vi "Main.vi"() -> ()   [LabVIEW 2020]
uses:
  System.Windows.Forms
  Global_Variable/Global.vi
  Database/Global1.vi
  <userlib>/_MGI/Menu Building/MenuTypes/MenuStrip/MGI_MenuStrip.lvclass
  <userlib>/_MGI/Menu Building/MenuItemStatusChange/MGI_MenuItemStatusChange.lvclass
  S7/S7.lvlib
panel:
  in  "Result":string[][](table)
  out "传感器码":string
  out "上序状态":string
  in  "Andon":enum32{"未选择", "缺料报警", "质量报警", "故障报警"}(radio)
  out "PLC":bool
  in  "菜单":refnum<k24>(container)
  out "逆向空载":bool
  out "试验计时":u16
  out "生产数量":i32
  out "合格数量":i32
  out "userStatus":string caption="用户状态"
  out "userName":string caption="用户名"
  out "connectionMode":string caption="联机类型"
  out "产品型号":string
  out "手柄开启力":bool
  out "手柄锁紧力":bool
  out "振动NVH":bool
  out "备用试验1":bool
  out "备用试验2":bool
  out "手柄保持力":bool caption="管柱保持力"
  out "锁紧/开启":bool
  out "手柄推拉力":bool caption="管柱推拉力"
  in  "更换产品":refnum<vi>
  out "提示信息":string
  out "错误":bool
  out "时间字符串":string
  out "日期字符串":string
  out "自动":bool
  # "滑移力检测"
  # "上序状态"
  # "试验项目"
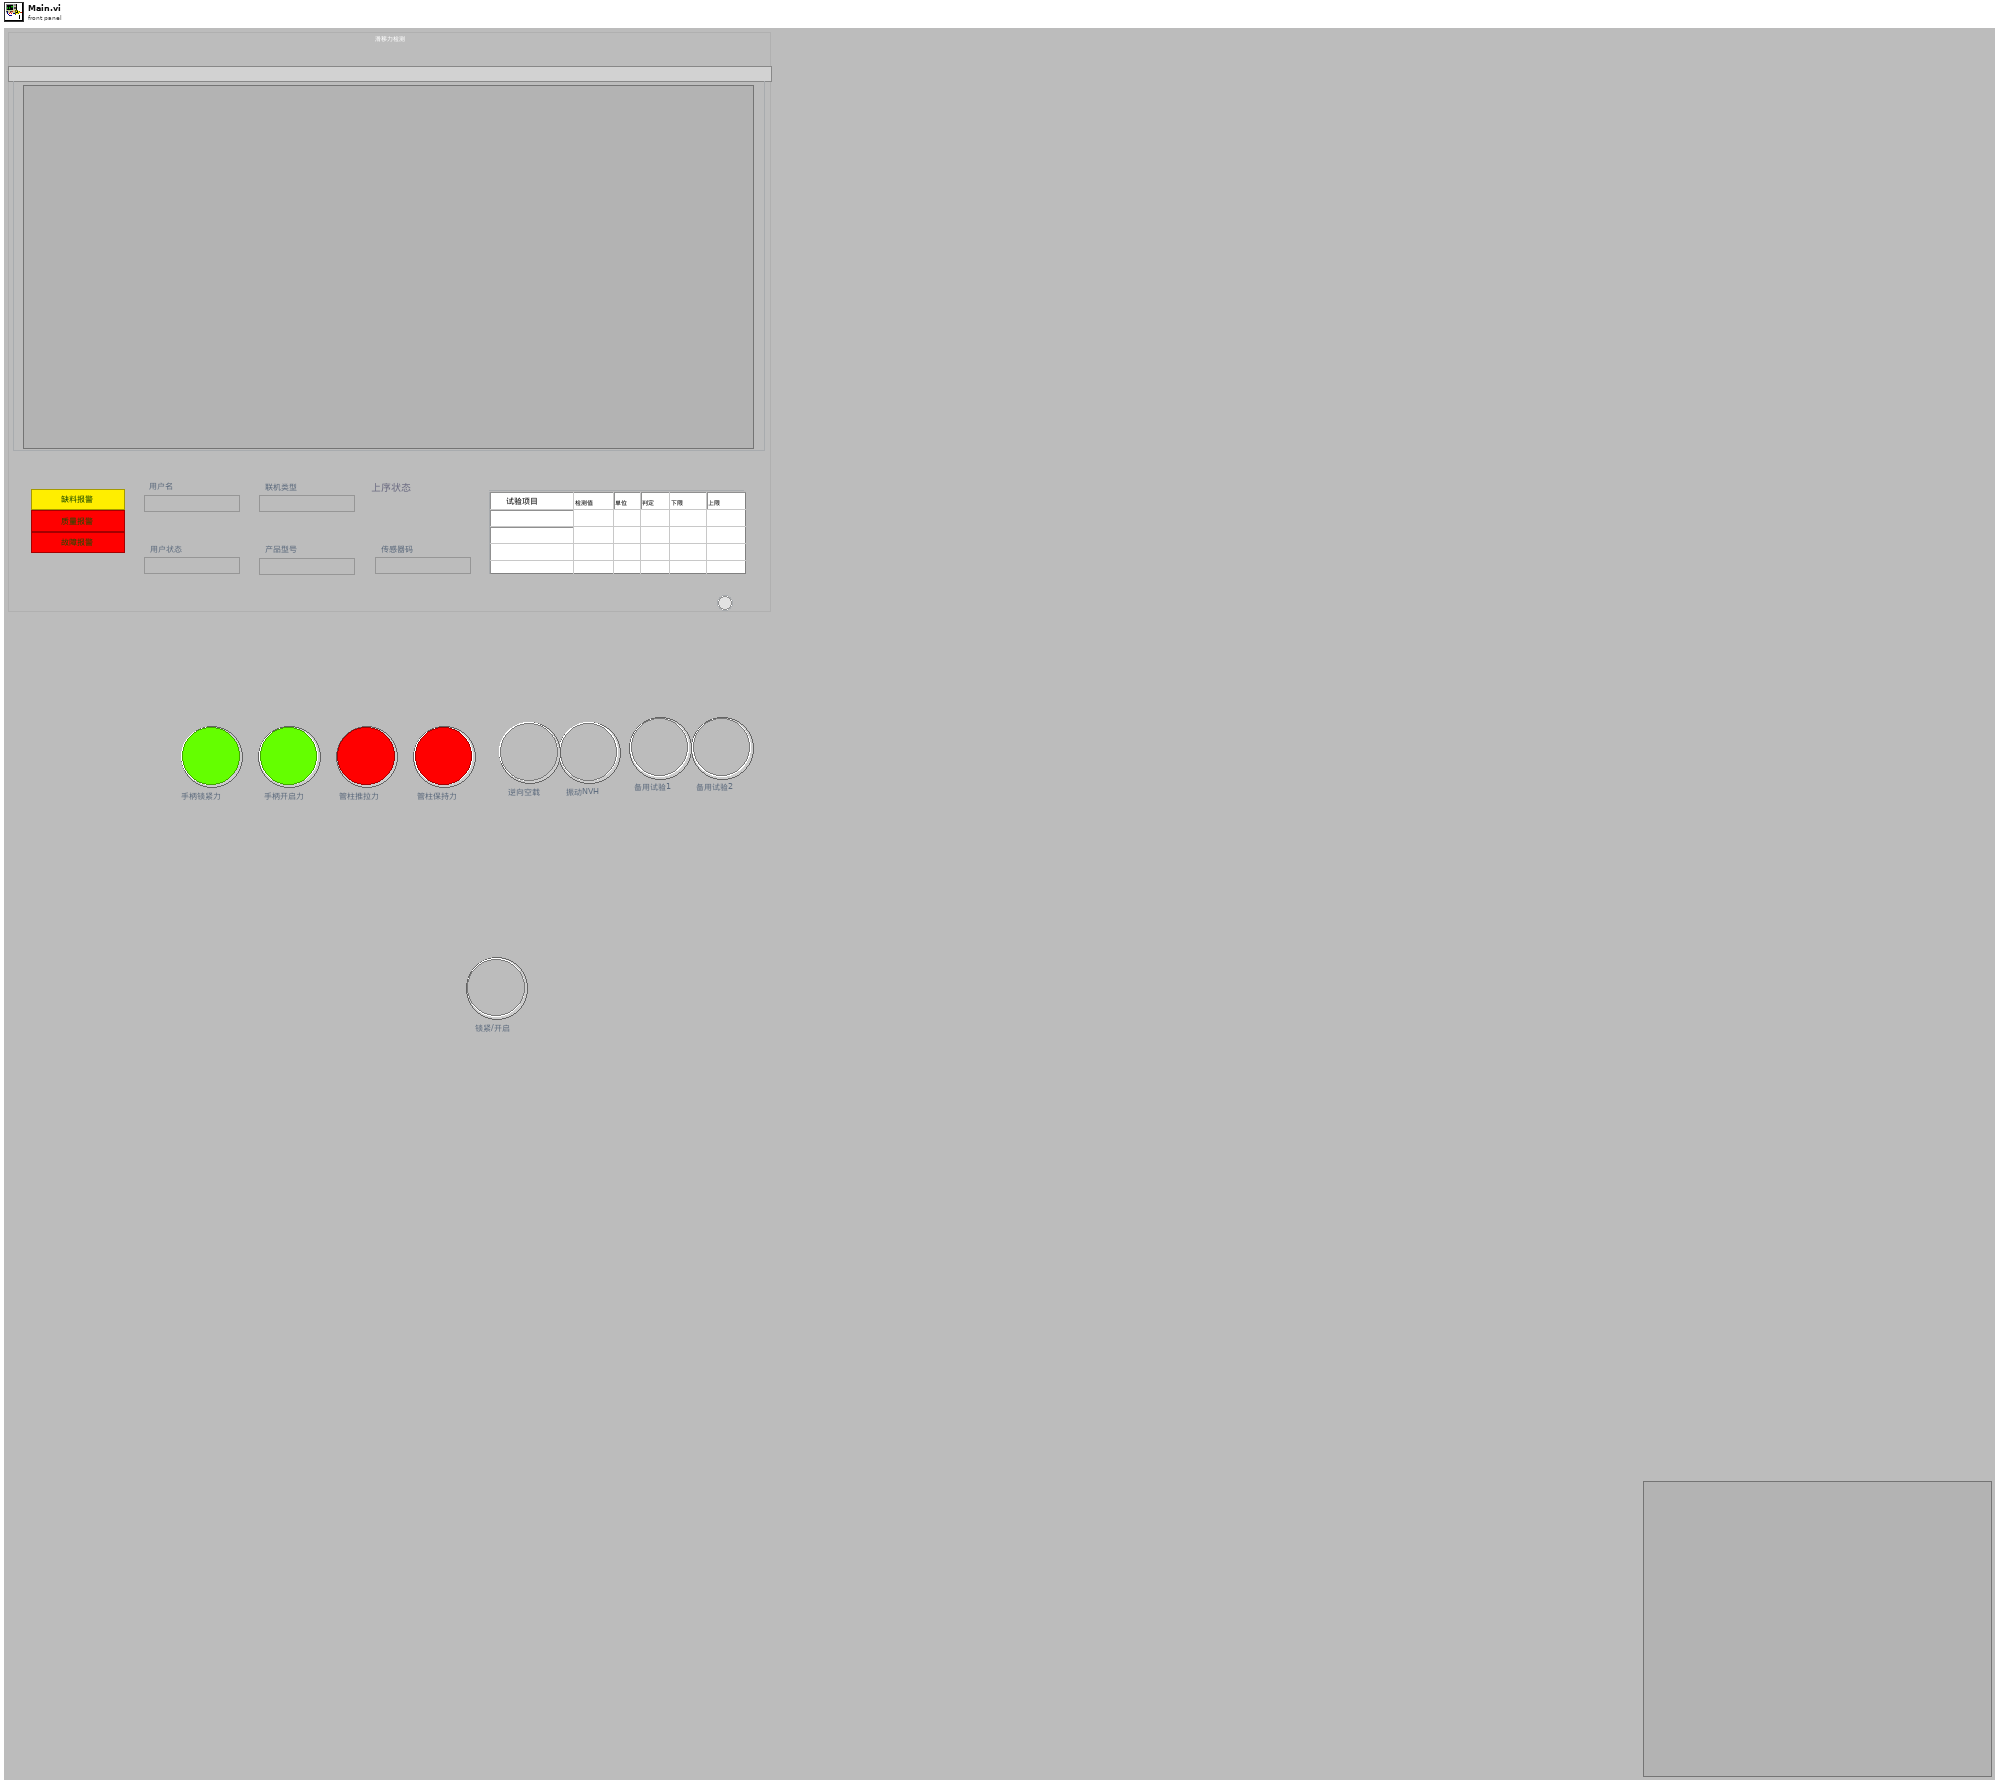
[diagram p1: front panel]
types:
  T1 = typedef "S7.lvlib/Broadcast Events--cluster.ctl" = cluster{"Module Did Init":refnum<user-event>, "Status Updated":refnum<user-event>, "Error Reported":refnum<user-event>, "Module Did Stop":refnum<user-event>, "Update Module Execution Status":refnum<user-event>}
  T2 = enum32{"Invalid", "Standard", "Closed", "Hidden", "Minimized", "Maximized"}
  T3 = cluster{"设备名称":string, "操作人员":string, "设备状态":enum16{"设备离线", "设备正常", "设备缺料", "设备故障", "质量报警"}, "附加信息":string}
  T4 = enum32{"invalid app kind", "Development System", "Run Time System", "Student Edition", "Embedded LabVIEW", "Evaluation", "Custom"}
  T5 = cluster{"用户编号":string, "用户名":string, "用户密码(密文)":string, "用户权限":string}
  T6 = cluster{"Core":cluster{"Current VI Reference":refnum<vi>, "Close Panel on Exit?":bool}, "Your Boolean data":bool, "Your string data":string}
  T7 = cluster{"Current VI Reference":refnum<vi>, "Close Panel on Exit?":bool}
  T8 = cluster{"设备名称":string, "用户名":string, "设备状态":enum16{"设备离线", "设备正常", "设备缺料", "设备故障", "质量报警"}, "附加信息":string}
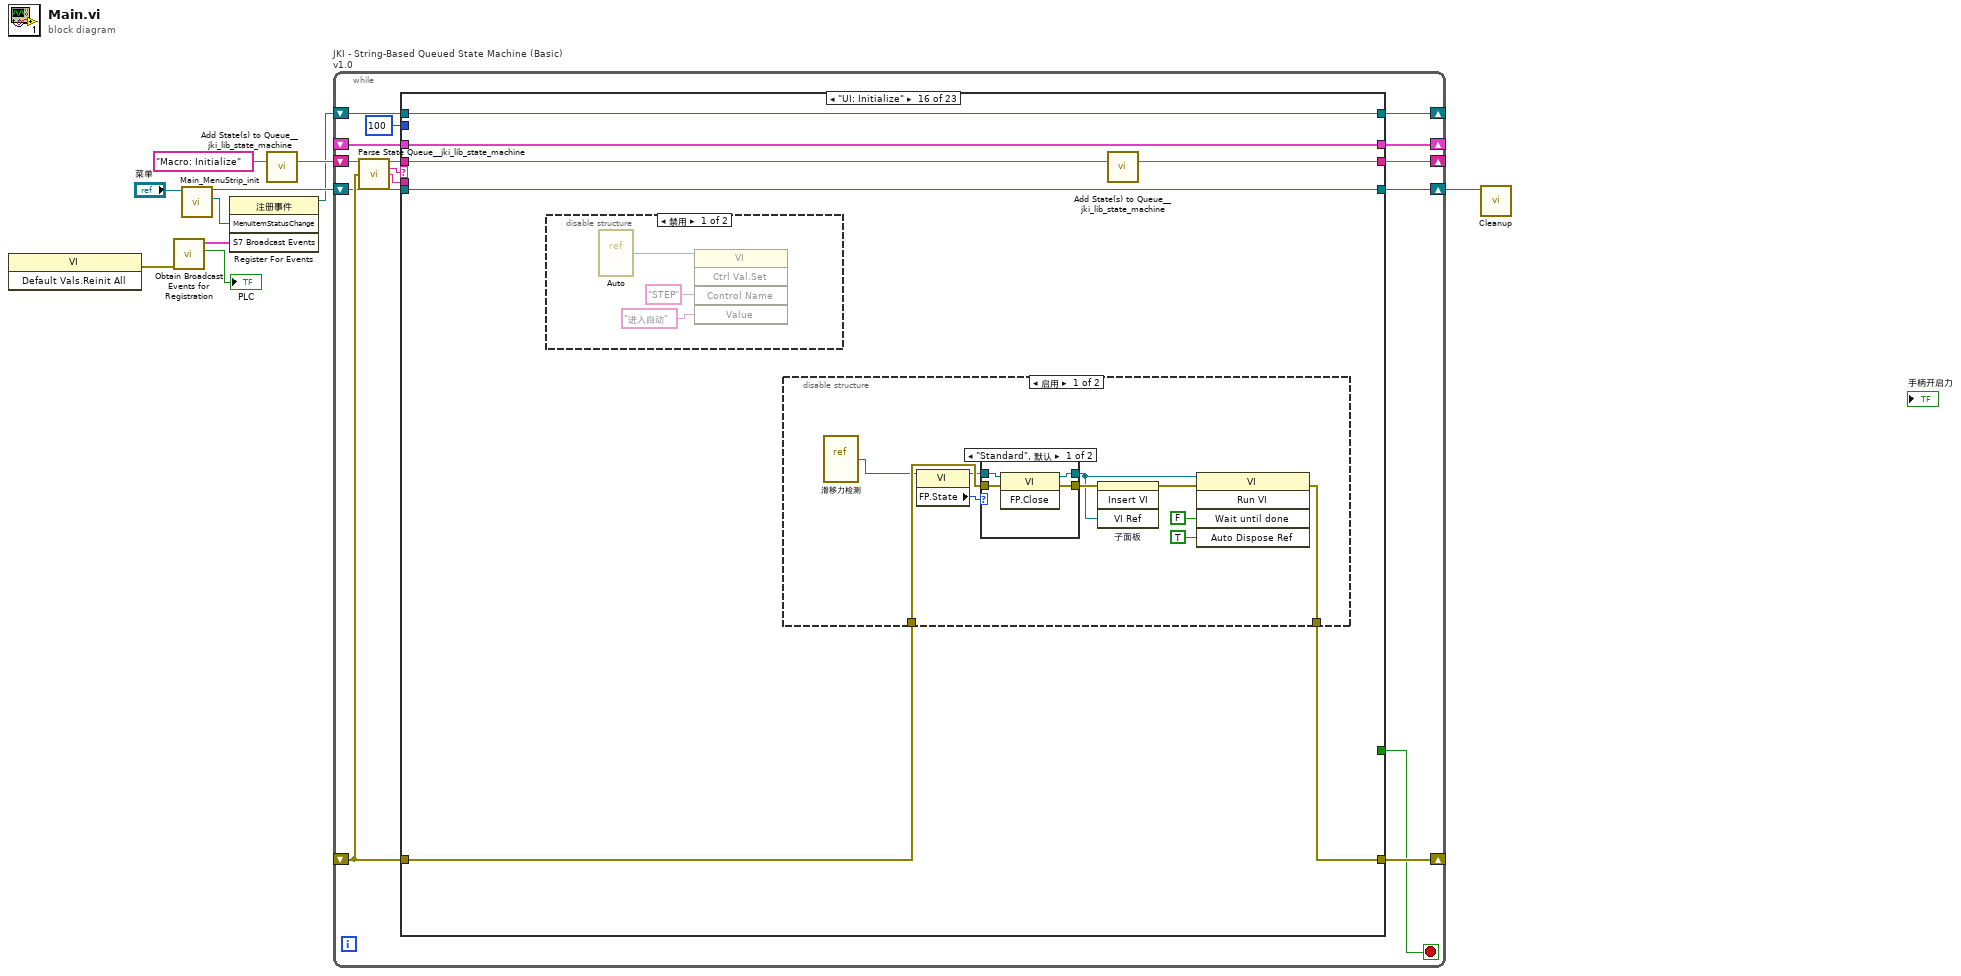
[diagram p0: block diagram]
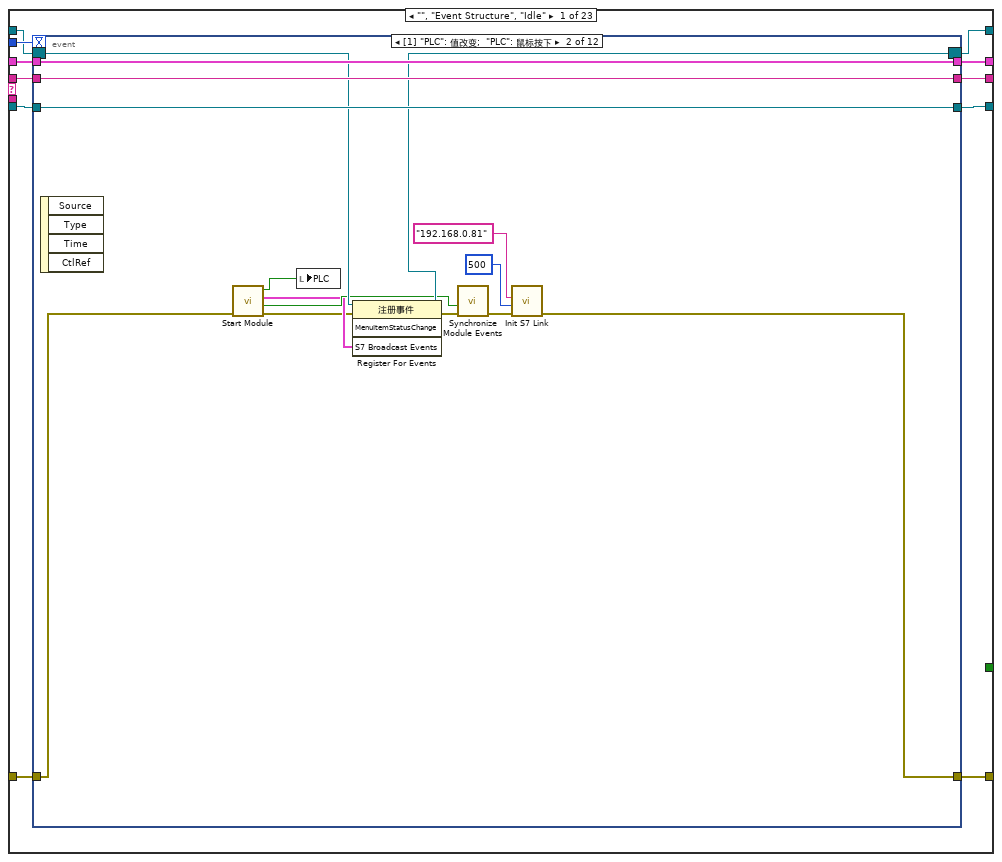
[diagram p2: hidden frame]
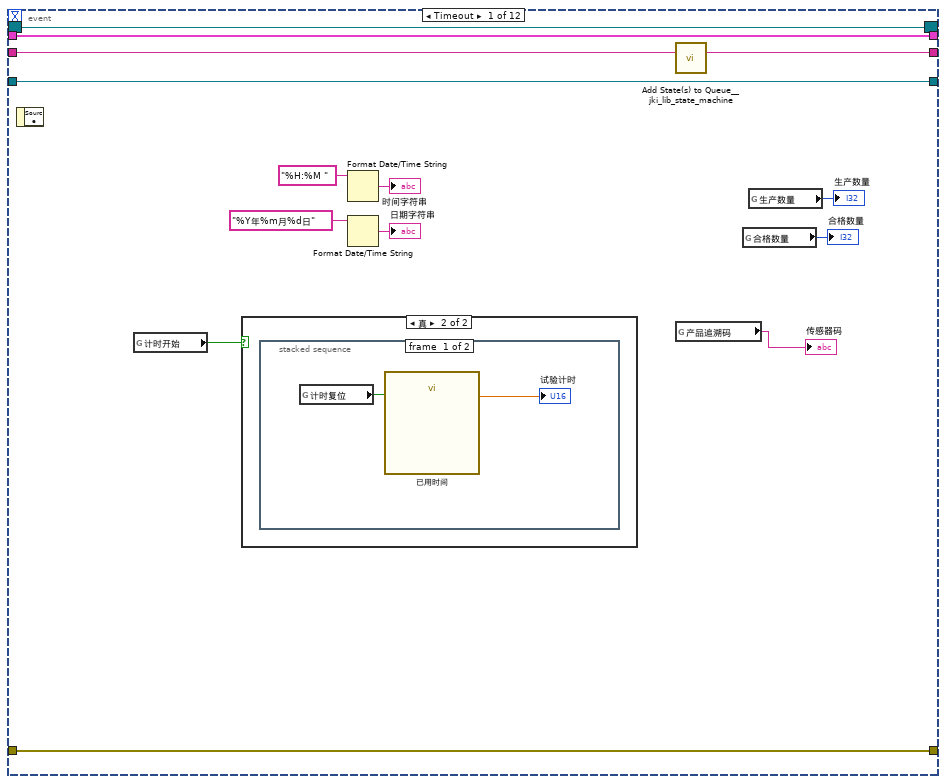
[diagram p3: hidden frame]
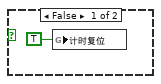
[diagram p4: hidden frame]
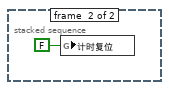
[diagram p5: hidden frame]
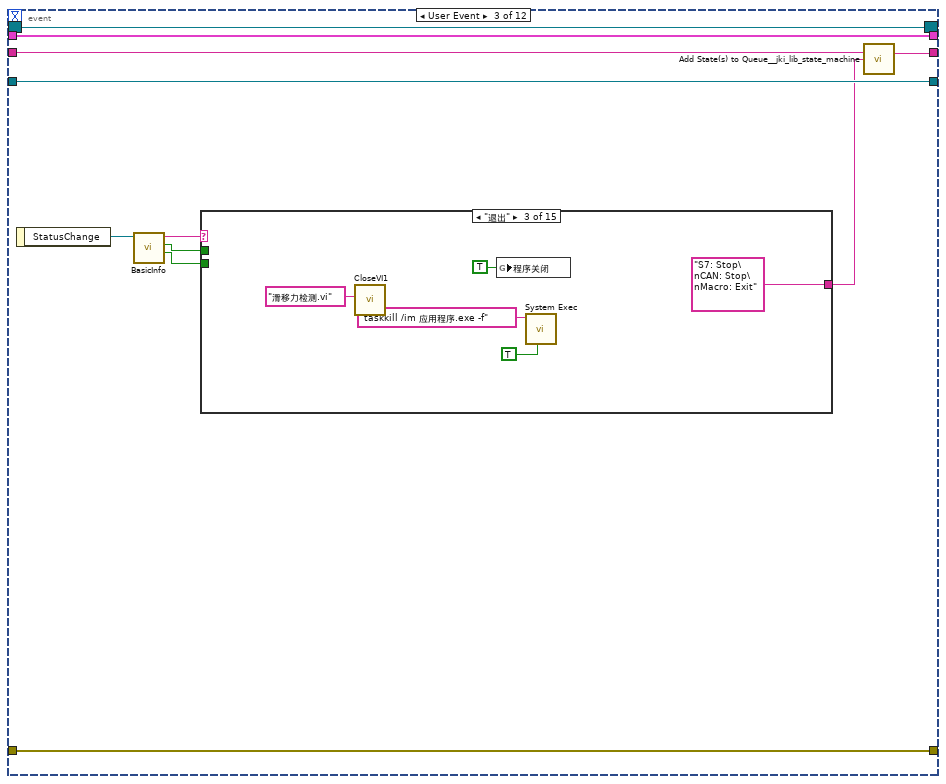
[diagram p6: hidden frame]
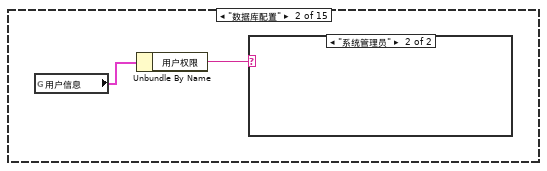
[diagram p8: hidden frame]
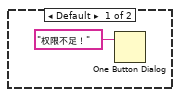
[diagram p9: hidden frame]
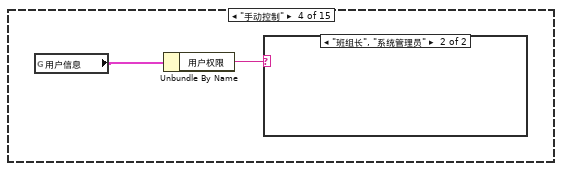
[diagram p10: hidden frame]
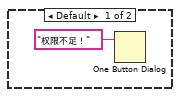
[diagram p11: hidden frame]
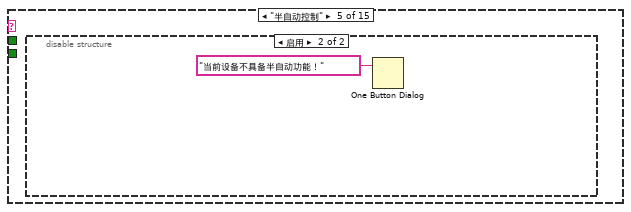
[diagram p12: hidden frame]
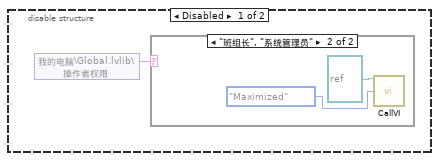
[diagram p13: hidden frame]
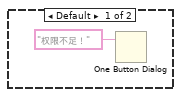
[diagram p14: hidden frame]
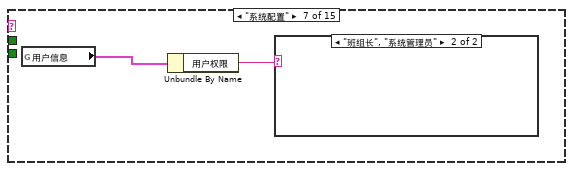
[diagram p16: hidden frame]
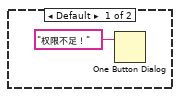
[diagram p17: hidden frame]
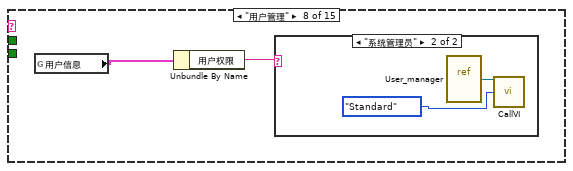
[diagram p18: hidden frame]
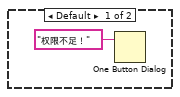
[diagram p19: hidden frame]
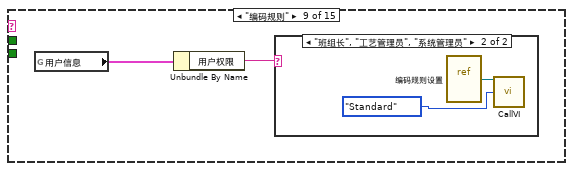
[diagram p20: hidden frame]
diagram:
  n1 = invoke class="VI" method="Default Vals.Reinit All"() -> (error out=w3:errorcluster)  [unwired: 3 in, 2 out]
  n2 = call "Obtain Broadcast Events for Registration.vi"("error in (no error)"=w3) -> ("Already running?"=→"PLC":bool, "S7 Broadcast Events"=w5:T1)  [unwired: 8 in, 1 out]
  n3 = call "Main_MenuStrip_init.vi"("MenuStrip"="菜单") -> ("MenuItemStatusChange"=w2:refnum<user-event>, "Menu out"=w7:refnum<class "MGI_MenuStrip.lvclass">)  [unwired: 9 in]
  n4 = register-events(w2, w5) -> (reference out=w1:refnum<event-registration>)  [unwired: 2 in, 1 out]
  n5 = call <vilib>:"Add State(s) to Queue__jki_lib_state_machine.vi"("State(s) in (\"\")"="Macro: Initialize") -> ("States Out"=w10:string)  [unwired: 14 in]
  n6 = while "JKI - String-Based Queued State Machine (Basic) v1.0" {
    shift-right: [w19] -> _
    shift-left: _ -> [w18]
    shift-right: [w21] -> _
    shift-left: _ -> [w16]
    shift-right: [w20] -> _
    shift-left: w10 -> [w22]
    shift-right: [w14] -> w6
    shift-left: w7 -> [w15]
    shift-right: [w12] -> _
    shift-left: w1 -> [w11]
    stop <- w13 stop-if-true
    n7 = call <vilib>:"Parse State Queue__jki_lib_state_machine.vi"("State Queue"=w22, "Error In (no error)"=w16) -> ("Remaining States"=w24:string, "Current State"=w25:string, "Arguments"=w23:string)  [unwired: 11 in]
    n8 = case shown="\"UI: Initialize\"" w25 {
      selector: w25 -> [_ _ w243 _ _ _ _ _ _ _ _ _ _ _ _ _ _ _ _ _ _ _ _]
      tunnel: w24 -> [w36 w240 w247 w267 w275 w282 w288 w292 w298 w304 w310 w319 w330 w338 w344 w351 w378 w417 w425 w438 w466 w473 w485]
      tunnel: w23 -> [_ _ _ _ _ _ _ _ _ _ _ _ _ _ _ _ _ _ w420 w432 _ _ _]
      tunnel: w18 -> [w34 w237 w245 w258 w272 w280 w285 w293 w301 w307 w313 w316 _ w333 w341 w349 w376 w414 w423 w434 w463 w470 w482]
      tunnel: [w33 w238 w249 w264 errorcluster {"status"=FALSE, "code"=0, "source"=""} ("error out") w279 w286 w290 w296 w303 w309 w317 w327 w334 w342 w348 w374 w415 w421 w435 w464 w471 w483] -> w21
      tunnel: w16 -> [w32 w238 w248 w264 w271 w279 w286 w290 w297 w303 w309 w317 w327 w335 w342 w345 w374 w415 w422 w436 w464 w471 w483]
      tunnel: [w35 w239 w246 w266 w274 w281 w287 w292 w299 w305 w311 w318 w329 w337 w343 w350 w377 w416 w424 w437 w465 w472 w484] -> w20
      tunnel: [w31 w237 w245 w265 w272 w280 w285 w293 w301 w307 w313 w316 w328 w333 w341 w349 w376 w414 w423 w434 w463 w470 w482] -> w19
      tunnel: 100 ("Timeout") -> [w30 _ _ _ _ _ _ _ _ _ _ _ _ _ _ _ _ _ _ _ _ _ _]
      tunnel: w15 -> [w29 w236 w242 w255 w269 w278 w284 w291 w300 w306 w312 w315 w321 w332 w340 w347 w375 w413 w419 w431 w462 w468 w475]
      tunnel: [w28 w236 w242 w255 w269 w278 w284 w291 w300 w306 w312 w315 w321 w332 w340 w347 w375 w413 w419 w431 w462 w468 w475] -> w14
      tunnel: [_ _ _ _ _ TRUE _ _ _ _ _ _ _ _ _ _ _ _ _ _ _ _ _] -> w13
      tunnel: [w26 w235 w241 w254 w268 w276 w283 w294 w295 w302 w308 w314 w322 w331 w339 w346 w373 w412 w418 w430 w461 w467 w474] -> w12
      tunnel: w11 -> [w27 w235 w241 w254 w268 w276 w283 w294 w295 w302 w308 w314 w322 w331 w339 w346 w373 w412 w418 w430 w461 w467 w474]
      frame "", "Event Structure", "Idle" {
        n9 = event shown="[1] \"PLC\": 值改变;  \"PLC\": 鼠标按下" {
          selector: w27 -> [w39 w64 w70 w127 w134 w141 w148 w162 w171 w176 w185 _]
          dyn-events: [w39 w63 w70 w127 w134 w141 w148 w162 w171 w176 w185 _] -> w26
          timeout: w30 -> [_ _ _ _ _ _ _ _ _ _ _ _]
          tunnel: w36 -> [w50 w68 w79 w128 w135 w144 w151 w159 w173 w183 w187 w229]
          tunnel: [w49 w68 w77 w129 w136 w145 w152 w160 w174 w182 w188 w229] -> w35
          tunnel: w34 -> [w48 w69 w78 w131 w139 w146 w153 w161 w175 w180 w190 w230]
          tunnel: [w40 w65 w80 w132 w137 w142 w154 w157 w172 w181 w189 w227] -> w33
          tunnel: w32 -> [w40 w66 w80 w132 w137 w142 w155 w157 w172 w181 w189 w227]
          tunnel: [w48 w69 w78 w131 w139 w146 w153 w161 w175 w180 w190 w230] -> w31
          tunnel: w29 -> [w38 w67 w73 w130 w138 w143 w150 w158 _ _ _ w228]
          tunnel: [w38 w67 w73 w130 w138 w143 w150 w158 _ _ _ w228] -> w28
          event Timeout {
            n10 = event-data() -> ()  [unwired: 1 in, 1 out]
            n11 = global read "Global.vi" "计时开始"() -> (w41:bool)
            n12 = case shown="真" w41 {
              frame False {
                n13 = global write "Global.vi" "计时复位"(TRUE ("计时复位")) -> ()
              }
              frame True {
                n14 = stacked-sequence {
                  frame #0 {
                    n15 = global read "Global.vi" "计时复位"() -> (w52:bool)
                    n16 = call "已用时间"("Reset"=w52) -> ("Elapsed Time (s)"=→"试验计时":dbl)  [unwired: 11 in, 7 out]
                  }
                  frame #1 {
                    n17 = global write "Global.vi" "计时复位"(FALSE ("计时复位")) -> ()
                  }
                }
              }
            }
            n18 = Format Date/Time String(time format string (%c)="%H:%M ") -> (date/time string=→"时间字符串":string)  [unwired: 2 in]
            n19 = Format Date/Time String(time format string (%c)="%Y年%m月%d日") -> (date/time string=→"日期字符串":string)  [unwired: 2 in]
            n20 = call <vilib>:"Add State(s) to Queue__jki_lib_state_machine.vi"("State(s) in (\"\")"=w50) -> ("States Out"=w49:string)  [unwired: 14 in]
            n21 = global read "Global.vi" "产品追溯码"() -> (→"传感器码":string)
            n22 = global read "Global.vi" "合格数量"() -> (→"合格数量":i32)
            n23 = global read "Global.vi" "生产数量"() -> (→"生产数量":i32)
          }
          event "PLC": Value Change; "PLC": Mouse Down {
            n24 = event-data() -> ()  [unwired: 1 in, 4 out]
            n25 = call "Start Module.vi"("error in (no error)"=w66) -> ("error out"=w57:errorcluster, "Wait for Event Sync?"=w62:bool, "S7 Broadcast Events"=w61:T1, "Module Was Already Running?"=w60:bool)  [unwired: 7 in]
            n26 = local write "PLC"(w60) -> ()
            n27 = register-events(reference=w64, error in=w57, w61) -> (reference out=w63:refnum<event-registration>, error out=w56:errorcluster)  [unwired: 1 in]
            n28 = call "Synchronize Module Events.vi"("error in (no error)"=w56, "Wait for Event Sync?"=w62) -> ("error out"=w55:errorcluster)  [unwired: 9 in]
            n29 = call "Init S7 Link.vi"("error in (no error)"=w55, "超时"=500, "IP"="192.168.0.81") -> ("error out"=w65:errorcluster)  [unwired: 8 in]
          }
          event User Event {
            n30 = event-data() -> ("StatusChange"=w71:refnum<class "MGI_MenuItemStatusChange.lvclass">)  [unwired: 1 in]
            n31 = call <userlib>:"BasicInfo.vi"("MGI_MenuItemStatusChange in"=w71) -> ("Enabled?"=w74:bool, "Checked?"=w75:bool, "Tag"=w76:string)  [unwired: 7 in, 1 out]
            n32 = case shown="\"退出\"" w76 {
              tunnel: w75 -> [_ _ _ _ _ _ _ _ _ _ _ _ _ _ _]
              tunnel: w74 -> [_ _ _ _ _ _ _ _ _ _ _ _ _ _ _]
              tunnel: [_ _ "S7: Stop\nCAN: Stop\nMacro: Exit" _ _ _ _ _ _ _ _ _ _ _ _] -> w72
              frame "假", Default {
              }
              frame "数据库配置" {
                n33 = global read "Global1.vi" "用户信息"() -> (w81:T5)
                n34 = Unbundle By Name(w81) -> ("用户权限"=w82:string)
                n35 = case shown="\"系统管理员\"" w82 {
                  frame Default {
                    n36 = One Button Dialog(message="权限不足！" ("消息")) -> ()  [unwired: 1 in, 1 out]
                  }
                  frame "系统管理员" {
                  }
                }
              }
              frame "退出" {
                n37 = call "CloseVI1.vi"("名称或相对路径"="滑移力检测.vi") -> ()  [unwired: 10 in, 1 out]
                n38 = global write "Global.vi" "程序关闭"(TRUE ("程序关闭")) -> ()
                n39 = call <vilib>:"System Exec.vi"("run minimized? (F)"=TRUE, "command line"="taskkill /im 应用程序.exe -f") -> ()  [unwired: 6 in, 4 out]
              }
              frame "手动控制" {
                n40 = global read "Global1.vi" "用户信息"() -> (w89:T5)
                n41 = Unbundle By Name(w89) -> ("用户权限"=w90:string)
                n42 = case shown="\"班组长\", \"系统管理员\"" w90 {
                  frame Default {
                    n43 = One Button Dialog(message="权限不足！" ("消息")) -> ()  [unwired: 1 in, 1 out]
                  }
                  frame "班组长", "系统管理员" {
                  }
                }
              }
              frame "半自动控制" {
                n44 = disable-structure shown="启用" {
                  frame Disabled {
                    n45 = shared-variable "我的电脑\\Global.lvlib\\操作者权限"() -> (w92:string)  [unwired: 1 in, 1 out]
                    n46 = case shown="\"班组长\", \"系统管理员\"" w92 {
                      frame Default {
                        n47 = One Button Dialog(message="权限不足！" ("消息")) -> ()  [unwired: 1 in, 1 out]
                      }
                      frame "班组长", "系统管理员" {
                        n48 = call "CallVI.vi"("VI引用"=refnum<vi> refnum, "状态"=T2."Maximized") -> ()  [unwired: 12 in, 2 out]
                      }
                    }
                  }
                  frame Enabled {
                    n49 = One Button Dialog(message="当前设备不具备半自动功能！" ("消息")) -> ()  [unwired: 1 in, 1 out]
                  }
                }
              }
              frame "产品管理" {
              }
              frame "系统配置" {
                n50 = global read "Global1.vi" "用户信息"() -> (w97:T5)
                n51 = Unbundle By Name(w97) -> ("用户权限"=w98:string)
                n52 = case shown="\"班组长\", \"系统管理员\"" w98 {
                  frame Default {
                    n53 = One Button Dialog(message="权限不足！" ("消息")) -> ()  [unwired: 1 in, 1 out]
                  }
                  frame "班组长", "系统管理员" {
                  }
                }
              }
              frame "用户管理" {
                n54 = global read "Global1.vi" "用户信息"() -> (w100:T5)
                n55 = Unbundle By Name(w100) -> ("用户权限"=w101:string)
                n56 = case shown="\"系统管理员\"" w101 {
                  frame Default {
                    n57 = One Button Dialog(message="权限不足！" ("消息")) -> ()  [unwired: 1 in, 1 out]
                  }
                  frame "系统管理员" {
                    n58 = vi-ref "User_manager.vi"() -> (w104:refnum<vi>)
                    n59 = call "CallVI.vi"("VI引用"=w104, "状态"=T2."Standard") -> ()  [unwired: 12 in, 2 out]
                  }
                }
              }
              frame "编码规则" {
                n60 = global read "Global1.vi" "用户信息"() -> (w105:T5)
                n61 = Unbundle By Name(w105) -> ("用户权限"=w106:string)
                n62 = case shown="\"班组长\", \"工艺管理员\", \"系统管理员\"" w106 {
                  frame Default {
                    n63 = One Button Dialog(message="权限不足！" ("消息")) -> ()  [unwired: 1 in, 1 out]
                  }
                  frame "班组长", "工艺管理员", "系统管理员" {
                    n64 = vi-ref "编码规则设置.vi"() -> (w109:refnum<vi>)
                    n65 = call "CallVI.vi"("VI引用"=w109, "状态"=T2."Standard") -> ()  [unwired: 12 in, 2 out]
                  }
                }
              }
              frame "易损件管理" {
                n66 = vi-ref "易损件管理.vi"() -> (w111:refnum<vi>)
                n67 = call "CallVI.vi"("VI引用"=w111, "状态"=T2."Standard") -> ()  [unwired: 12 in, 2 out]
              }
              frame "物料批次管理" {
                n68 = vi-ref "批次管理.vi"() -> (w113:refnum<vi>)
                n69 = call "CallVI.vi"("VI引用"=w113, "状态"=T2."Standard") -> ()  [unwired: 12 in, 2 out]
              }
              frame "报表" {
                n70 = call "文件对话框"("start path"=path "D:/report", "prompt"="打开报表", "pattern (all files)"="*.doc;*.docx", "pattern label"="Word 文档") -> ("selected path"=w114:path, "error out"=w115:errorcluster)  [unwired: 8 in, 2 out]
                n71 = case shown="无错误" w115 {
                  selector: w115 -> [w121 w123]
                  tunnel: w114 -> [w122 _]
                  frame No Error {
                    w120 = 1 items=["Normal", "Maximize", "Minimize"] ("cpubbs_WindowState")
                    n72 = call "Open_Word.vi"("File Path"=w122, "cpubbs_WindowState"=w120, "错误输入（无错误）"=w121) -> ()  [unwired: 12 in, 1 out]
                  }
                  frame Error {
                    n73 = call <vilib>:"Clear Errors.vi"("error in (no error)"=w123) -> ()  [unwired: 5 in, 2 out]
                  }
                }
              }
              frame "报警信息" {
              }
              frame "关于" {
              }
              frame "操作演示" {
                n74 = call <vilib>:"Application Directory.vi"() -> ("Application Directory"=w126:path)
                n75 = Build Path(base path=w126, name or relative path="操作演示" ("名称或相对路径")) -> (appended path=w125:path)
                n76 = call "自动播放ppt.vi"("路径"=w125) -> ()  [unwired: 10 in, 1 out]
              }
            }
            n77 = call <vilib>:"Add State(s) to Queue__jki_lib_state_machine.vi"("State(s) in (\"\")"=w79, "State(s) at Back (\"\")"=w72) -> ("States Out"=w77:string)  [unwired: 13 in]
          }
          event User Event {
            n78 = event-data() -> ("Init?"=w133:bool)  [unwired: 1 in, 1 out]
            n79 = local write "PLC"(w133) -> ()
            n80 = call <vilib>:"Add State(s) to Queue__jki_lib_state_machine.vi"("State(s) in (\"\")"=w128) -> ("States Out"=w129:string)  [unwired: 14 in]
          }
          event User Event {
            n81 = event-data() -> ("Running?"=w140:bool)  [unwired: 1 in]
            n82 = local write "PLC"(w140) -> ()
            n83 = call <vilib>:"Add State(s) to Queue__jki_lib_state_machine.vi"("State(s) in (\"\")"=w135) -> ("States Out"=w136:string)  [unwired: 14 in]
          }
          event User Event {
            n84 = event-data() -> ()  [unwired: 1 in, 7 out]
            n85 = local write "PLC"(FALSE ("PLC")) -> ()
            n86 = call <vilib>:"Add State(s) to Queue__jki_lib_state_machine.vi"("State(s) in (\"\")"=w144) -> ("States Out"=w145:string)  [unwired: 14 in]
          }
          event User Event {
            n87 = event-data() -> ("Error"=w156:errorcluster)  [unwired: 1 in]
            n88 = Merge Errors(w156, w155) -> (w154:errorcluster)
            n89 = call <vilib>:"Add State(s) to Queue__jki_lib_state_machine.vi"("State(s) in Front (\"\")"="S7: Initialize\nIdle", "State(s) in (\"\")"=w151) -> ("States Out"=w152:string)  [unwired: 13 in]
          }
          event "自动": Mouse Down {
            n90 = event-data() -> ()  [unwired: 1 in, 1 out]
            n91 = disable-structure shown="禁用" {
              frame Disabled {
                n92 = local read "自动"() -> (w163:bool)
                n93 = case shown="假" w163 {
                  frame False {
                    n94 = call "设备状态.vi"() -> ("Status_Read"=w164:i16)  [unwired: 11 in]
                    n95 = case shown="5" w164 {
                      frame 0, Default {
                        n96 = One Button Dialog(message="请复位！" ("消息")) -> ()  [unwired: 1 in, 1 out]
                      }
                      frame 5 {
                      }
                    }
                  }
                  frame True {
                    n97 = Two Button Dialog(message="确定要退出自动？" ("消息")) -> (T button?=w166:bool)  [unwired: 2 in]
                    n98 = case shown="真" w166 {
                      frame False {
                      }
                      frame True {
                        n99 = vi-ref "Auto.vi"() -> (w170:refnum<vi>)
                        n100 = invoke class="VI" method="Ctrl Val.Set"(reference=w170, "Control Name"="STEP" ("控件名"), "Value"="退出自动" ("控件名")) -> ()  [unwired: 2 in, 5 out]
                      }
                    }
                  }
                }
              }
              frame Enabled {
              }
            }
            n101 = call <vilib>:"Add State(s) to Queue__jki_lib_state_machine.vi"("State(s) in (\"\")"=w159) -> ("States Out"=w160:string)  [unwired: 14 in]
          }
          event "错误": Mouse Down {
            n102 = event-data() -> ()  [unwired: 1 in, 8 out]
            n103 = call <vilib>:"Add State(s) to Queue__jki_lib_state_machine.vi"("State(s) in (\"\")"=w173) -> ("States Out"=w174:string)  [unwired: 14 in]
          }
          event Panel Close? {
            n104 = event-data() -> ()  [unwired: 1 in, 1 out]
            n105 = global write "Global.vi" "程序关闭"(TRUE ("程序关闭")) -> ()
            n106 = call <vilib>:"Add State(s) to Queue__jki_lib_state_machine.vi"("State(s) in Front (\"\")"="S7: Stop\nMacro: Exit", "State(s) in (\"\")"=w183) -> ("States Out"=w182:string)  [unwired: 13 in]
            n107 = event-data("Discard?"=TRUE) -> ()  [unwired: 1 in, 1 out]
          }
          event "更换产品": Value Change {
            n108 = event-data() -> ("NewVal"=w186:refnum<vi>)  [unwired: 1 in, 5 out]
            n109 = stacked-sequence {
              tunnel: w186 -> [w192]
              tunnel: [w191] -> w184
              frame #0 {
                n110 = stacked-sequence {
                  tunnel: w192 -> [w193 _ _]
                  tunnel: [_ w196 _] -> w191
                  frame #0 {
                    n111 = disable-structure shown="禁用" {
                      disable-tunnel: w193 -> [w195 _]
                      frame Disabled {
                        n112 = control-ref of="子面板"() -> (w194:refnum<vi>)
                        n113 = call "Call_SubPanal.vi"("VI引用句柄"=w195, "SubPnl引用句柄"=w194) -> ()  [unwired: 9 in, 1 out]
                      }
                      frame Enabled {
                      }
                    }
                  }
                  frame #1 {
                    n114 = global read "Global.vi" "启用CAN"() -> (w197:bool)
                    n115 = case shown="假" w197 {
                      tunnel: ["CAN: Stop" "CAN: Stop\nIdle\nCAN: Start"] -> w196
                      frame False {
                      }
                      frame True {
                      }
                    }
                  }
                  frame #2 {
                    n116 = control-ref of="锁紧/开启"() -> (w200:refnum<vi>)
                    n117 = control-ref of="手柄保持力"() -> (w201:refnum<vi>)
                    n118 = control-ref of="手柄锁紧力"() -> (w202:refnum<vi>)
                    n119 = control-ref of="手柄开启力"() -> (w203:refnum<vi>)
                    n120 = control-ref of="手柄推拉力"() -> (w204:refnum<vi>)
                    n121 = global read "Global.vi" "试验项目"() -> (w207:bool[])
                    n122 = Build Array(w202, w203, w204, w201, w200) -> (w206:refnum<vi>[])
                    n123 = for {
                      tunnel: w206 -> [w211] mode=indexing
                      tunnel: w207 -> [w212] mode=indexing
                      shift-right: [w208] -> _
                      shift-left: 2000 -> [w209]
                      i -> [w210]
                      n124 = case shown="真" w212 {
                        tunnel: w211 -> [w213 w221]
                        tunnel: w210 -> [_ _]
                        tunnel: w209 -> [w215 w218]
                        tunnel: [w215 w216] -> w208
                        frame False {
                          n125 = property class="Bool (严格)"(reference=w213, "Top"=2000) -> ()  [unwired: 1 in, 2 out]
                        }
                        frame True {
                          n126 = Add(x=w218, y=130) -> (x+y=w216:i32)
                          n127 = Bundle(w216, 1250) -> (w219:cluster{i32, i32})  [unwired: 1 in]
                          n128 = property class="Bool (严格)"(reference=w221, "Position"=w219) -> ()  [unwired: 1 in, 2 out]
                        }
                      }
                    }
                  }
                }
              }
            }
            n129 = call <vilib>:"Add State(s) to Queue__jki_lib_state_machine.vi"("State(s) in Front (\"\")"=w184, "State(s) in (\"\")"=w187) -> ("States Out"=w188:string)  [unwired: 13 in]
          }
          event "Andon": Value Change {
            n130 = event-data() -> ("NewVal"=w226:enum32{"未选择", "缺料报警", "质量报警", "故障报警"})  [unwired: 1 in]
            n131 = case shown="\"缺料报警\"" w226 {
              tunnel: [enum16{"设备离线", "设备正常", "设备缺料", "设备故障", "质量报警"}."设备正常" ("设备状态") enum16{"设备离线", "设备正常", "设备缺料", "设备故障", "质量报警"}."设备缺料" ("设备状态") enum16{"设备离线", "设备正常", "设备缺料", "设备故障", "质量报警"}."质量报警" ("设备状态") enum16{"设备离线", "设备正常", "设备缺料", "设备故障", "质量报警"}."设备故障" ("设备状态")] -> w224
              frame "未选择", Default {
              }
              frame "缺料报警" {
              }
              frame "质量报警" {
              }
              frame "故障报警" {
              }
            }
            n132 = local read "userName"() -> (w223:string)
            n133 = Bundle By Name(cluster=T3 {"设备名称"="滑移力检测", "操作人员"="", "设备状态"=enum."设备离线", "附加信息"=""} ("设备信息"), "操作人员"=w223, "设备状态"=w224) -> (w222:T3)
            n134 = call "Change_Client.vi"("设备信息"=w222) -> ()  [unwired: 10 in, 1 out]
          }
        }
      }
      frame "---------- Core ----------" {
        n135 = call <vilib>:"Add State(s) to Queue__jki_lib_state_machine.vi"("State(s) in (\"\")"=w240) -> ("States Out"=w239:string)  [unwired: 14 in]
      }
      frame Default {
        w252 = 42 items=["No error", "Argument error", "Memory is full", "Out of zone", "End of file", "File already open", "Generic file I/O error", "File not found", "File permission error", "Disk is full", "Duplicate path", "Too many files open", "System feature not enabled", "Resource file not found", "Cannot add resource", "Resource not found", "Image not found", "Image memory error", "Pen does not exist", "Config type invalid", "Config token not found", "Config parse error", "Config memory error", "Bad external code format", "Bad external code offset", "External code not present", "Null window", "Destroy window error", "Null menu", "Print aborted", "Bad print record", "Print driver error", "Windows error during printing", "Memory error during printing", "Print dialog error", "Generic print error", "Invalid device refnum", "Device not found", "Device parameter error", "Device unit error", "Cannot open device", "Device call aborted", "Generic error", "Cancelled by user", "Object ID too low", "Object ID too high", "Object not in heap", "Unknown heap", "Unknown object (invalid DefProc)", "Unknown object (DefProc not in table)", "Message out of range", "Invalid (null) method", "Unknown message", "Manager call not supported", "Bad address", "Network operation in progress", "Network operation timed out", "Connection is busy", "Network attribute not supported", "Network error", "Address in use", "System out of memory", "Connection aborted", "Connection refused", "Not connected", "Already connected", "Connection closed", "Initialization error (interapplication manager)", "Bad occurrence", "Wait on unbound occurrence handler", "Occurrence queue overflow", "Datalog type conflict", "Unused", "Unrecognized type (interapplication manager)", "Memory corrupt", "Failed to make temporary DLL", "Old CIN version", "Drag socket not found", "Failed to load drop-object", "Failed to register OLE object", "Failed to release OLE object", "Format specifier type mismatch", "Unknown format specifier", "Too few format specifiers", "Too many format specifiers", "Scan failed", "Newer CIN version", "Error converting to variant", "Runtime menu error", "Password tampered", "Variant attribute not found", "Incompatible variant data type", "Event data is not available", "Event Store is not present", "Occurrence is not found", "Event Queue is not created", "Event info is not available", "Refnum passed is NULL", "Error retrieving Class GUID", "Error retrieving CoClass GUID", "Error retrieving TypeLib GUID.", "Bad built application magic bytes.", "Specific driver is different from the specific driver associated with the Logical Name.", "There is no session opened to the class driver.", "Max Error", "MAX - Error with config objects", "MAX - Error loading configuration", "MAX - Group not supported"]
        # "Current State"
        n136 = Format Into String(format string="Software Exception: Unhandled State \"%s\"." ("message"), error in=w248, w243) -> (resulting string=w251:string, error out=w250:errorcluster)  [unwired: 1 in]
        n137 = call <vilib>:"Error Cluster From Error Code.vi"("show call chain? (False)"=TRUE, "error in (no error)"=w250, "error message (\"\")"=w251, "error code (0)"=w252) -> ("error out"=w249:errorcluster)  [unwired: 5 in]
        n138 = call <vilib>:"Add State(s) to Queue__jki_lib_state_machine.vi"("State(s) in (\"\")"=w247) -> ("States Out"=w246:string)  [unwired: 14 in]
      }
      frame "Initialize Core Data" {
        # "originally closed?"
        # "exe?"
        n139 = property class="VI"() -> ("Front Panel.Open"=w263:bool)  [unwired: 2 in, 2 out]
        n140 = property class="App"() -> ("App.Kind"=w262:T4)  [unwired: 2 in, 2 out]
        n141 = control-ref of="Current VI Reference"() -> (w256:refnum<vi>)
        n142 = Not(x=w263) -> (.not. x?=w260:bool)
        n143 = Equal?(x=w262, y=T4."Run Time System" ("Application:Kind")) -> (x = y?=w259:bool)
        n144 = Or(x=w260, y=w259) -> (x .or. y?=w257:bool)
        n145 = Bundle By Name(cluster=w258, "Core.Current VI Reference"=w256, "Core.Close Panel on Exit?"=w257) -> (w265:T6)
        n146 = call <vilib>:"Add State(s) to Queue__jki_lib_state_machine.vi"("State(s) in (\"\")"=w267) -> ("States Out"=w266:string)  [unwired: 14 in]
      }
      frame "Error Handler" {
        n147 = call <vilib>:"General Error Handler.vi"("error in (no error)"=w271) -> ()  [unwired: 10 in, 5 out]
        n148 = call <vilib>:"Add State(s) to Queue__jki_lib_state_machine.vi"("State(s) in Front (\"\")"="/* Post Error States", "State(s) in (\"\")"=w275) -> ("States Out"=w274:string)  [unwired: 13 in]
      }
      frame "Exit" {
        n149 = call <vilib>:"Add State(s) to Queue__jki_lib_state_machine.vi"("State(s) in (\"\")"=w282) -> ("States Out"=w281:string)  [unwired: 14 in]
        n150 = Quit LabVIEW() -> ()  [unwired: 1 in]
      }
      frame "--------- Library --------" {
        n151 = call <vilib>:"Add State(s) to Queue__jki_lib_state_machine.vi"("State(s) in (\"\")"=w288) -> ("States Out"=w287:string)  [unwired: 14 in]
      }
      frame "S7: Initialize" {
        n152 = property on="PLC" class="Bool (严格)"("Val(Sgnl)"=FALSE ("值(信号)")) -> ()  [unwired: 2 in, 2 out]
      }
      frame "S7: Stop" {
        n153 = call "Stop Module.vi"("error in (no error)"=w297) -> ("error out"=w296:errorcluster)  [unwired: 10 in]
        n154 = call <vilib>:"Add State(s) to Queue__jki_lib_state_machine.vi"("State(s) in (\"\")"=w298) -> ("States Out"=w299:string)  [unwired: 14 in]
      }
      frame "CAN: Start" {
        n155 = call <vilib>:"Add State(s) to Queue__jki_lib_state_machine.vi"("State(s) in (\"\")"=w304) -> ("States Out"=w305:string)  [unwired: 14 in]
      }
      frame "CAN: Stop" {
        n156 = call <vilib>:"Add State(s) to Queue__jki_lib_state_machine.vi"("State(s) in (\"\")"=w310) -> ("States Out"=w311:string)  [unwired: 14 in]
      }
      frame "---------- Data ----------" {
        n157 = call <vilib>:"Add State(s) to Queue__jki_lib_state_machine.vi"("State(s) in (\"\")"=w319) -> ("States Out"=w318:string)  [unwired: 14 in]
      }
      frame "Data: Initialize" {
        w324 = T7 {"Current VI Reference"=refnum, "Close Panel on Exit?"=FALSE}  # Core
        w326 = TRUE  # Your Boolean data
        w325 = ""  # Your string data
        n158 = global write "Global.vi" "程序关闭"(FALSE ("程序关闭")) -> ()
        n159 = global write "Global.vi" "计时开始"(FALSE ("计时结束")) -> ()
        n160 = Bundle("Core"=w324, "Your Boolean data"=w326, "Your string data"=w325) -> (w328:T6)  [unwired: 1 in]
        n161 = call <vilib>:"Add State(s) to Queue__jki_lib_state_machine.vi"("State(s) in (\"\")"=w330) -> ("States Out"=w329:string)  [unwired: 14 in]
      }
      frame "Data: Cleanup" {
        n162 = Unbundle By Name(w333) -> ("Core.Current VI Reference"=w336:refnum<vi>)
        n163 = Close Reference(reference=w336, error in (no error)=w335) -> (error out=w334:errorcluster)
        n164 = call <vilib>:"Add State(s) to Queue__jki_lib_state_machine.vi"("State(s) in (\"\")"=w338) -> ("States Out"=w337:string)  [unwired: 14 in]
      }
      frame "---------- UI ----------" {
        # "Do not put any code in this frame.\n(It is a separator no-op. You can make a copy of this frame to create a new UI frame)"
        n165 = call <vilib>:"Add State(s) to Queue__jki_lib_state_machine.vi"("State(s) in (\"\")"=w344) -> ("States Out"=w343:string)  [unwired: 14 in]
      }
      frame "UI: Initialize" {
        n166 = disable-structure shown="禁用" {
          frame Disabled {
            n167 = vi-ref "Auto.vi"() -> (w354:refnum<vi>)
            n168 = invoke class="VI" method="Ctrl Val.Set"(reference=w354, "Control Name"="STEP" ("控件名"), "Value"="进入自动" ("控件名")) -> ()  [unwired: 2 in, 5 out]
          }
          frame Enabled {
          }
        }
        n169 = disable-structure shown="启用" {
          disable-tunnel: [w361 _] -> w348
          disable-tunnel: w345 -> [w360 _]
          frame Enabled {
            n170 = vi-ref "滑移力检测.vi"() -> (w355:refnum<vi>)
            n171 = property class="VI"(reference=w355) -> (reference out=w359:refnum<vi>, "FP.State"=w358:T2)  [unwired: 1 in, 1 out]
            n172 = case shown="\"Standard\", 默认" w358 {
              tunnel: w360 -> [w367 w369]
              tunnel: w359 -> [w368 w370]
              tunnel: [w366 w370] -> w356
              tunnel: [w365 w369] -> w357
              frame "Standard", Default {
                n173 = invoke class="VI" method="FP.Close"(reference=w368, error in=w367) -> (reference out=w366:refnum<vi>, error out=w365:errorcluster)  [unwired: 1 in, 1 out]
              }
              frame "Invalid", "Closed" {
              }
            }
            n174 = invoke on="子面板" class="SubPnl" method="Insert VI"(error in=w357, "VI Ref"=w356) -> (error out=w364:errorcluster)  [unwired: 2 in, 3 out]
            n175 = invoke class="VI" method="Run VI"(reference=w356, error in=w364, "Wait until done"=FALSE ("结束前等待"), "Auto Dispose Ref"=TRUE ("自动销毁引用")) -> (error out=w361:errorcluster)  [unwired: 1 in, 4 out]
          }
          frame Disabled {
            n176 = vi-ref "Auto.vi"() -> (w372:refnum<vi>)
            n177 = call "CallVI.vi"("VI引用"=w372, "状态"=T2."Maximized") -> ()  [unwired: 12 in, 2 out]
          }
        }
        n178 = call <vilib>:"Add State(s) to Queue__jki_lib_state_machine.vi"("State(s) in (\"\")"=w351) -> ("States Out"=w350:string)  [unwired: 14 in]
      }
      frame "UI: Init" {
        n179 = stacked-sequence {
          tunnel: w374 -> [_ _ _ _]
          frame #0 {
            n180 = global write "Global.vi" "程序关闭"(FALSE ("程序关闭")) -> ()
            n181 = global read "Global1.vi" "产品型号"() -> (w380:string)
            n182 = control-ref of="产品型号"() -> (w379:refnum<vi>)
            n183 = local write "产品型号"(w380) -> ()
            n184 = control-ref of="上序状态"() -> (w381:refnum<vi>)
            n185 = global write "Global.vi" "产品型号引用"(w379) -> ()
            n186 = global write "Global.vi" "上序状态颜色"(w381) -> ()
          }
          frame #1 {
            (unwired) "   " ("工位追溯码")
            w390 = 0
            n187 = global read "Global.vi" "上序状态颜色"() -> (w386:refnum<vi>)
            n188 = global write "Global.vi" "生产数量"(w390) -> ()
            n189 = global write "Global.vi" "合格数量"(w390) -> ()
            n190 = global read "Global1.vi" "用户信息"() -> (w384:T5)
            n191 = global read "Global1.vi" "联机模式"() -> (w383:enum16{"单机", "追溯"})
            n192 = property class="Str"(reference=w386, "Value"="" ("值")) -> ()  [unwired: 1 in, 2 out]
            n193 = Unbundle By Name(w384) -> ("用户名"=→"userName":string, "用户权限"=→"userStatus":string)
            n194 = case shown="\"追溯\"" w383 {
              tunnel: ["联网" ("connectionMode") "单机" ("connectionMode")] -> w391
              frame "追溯" {
              }
              frame "单机", Default {
              }
            }
            "connectionMode" <- w391
            "产品型号" <- "" ("产品型号")
          }
          frame #2 {
            n195 = control-ref of="提示信息"() -> (w395:refnum<vi>)
            n196 = control-ref of="自动"() -> (w396:refnum<vi>)
            n197 = control-ref of="错误"() -> (w397:refnum<vi>)
            n198 = control-ref of="Result"() -> (w398:refnum<vi>)
            n199 = control-ref of="更换产品"() -> (w394:refnum<vi>)
            n200 = global write "Global.vi" "提示信息"(w395) -> ()
            n201 = global write "Global.vi" "程序自动"(w396) -> ()
            n202 = global write "Global.vi" "报警图标"(w397) -> ()
            n203 = global write "Global.vi" "Result"(w398) -> ()
            n204 = global write "Global.vi" "更换产品"(w394) -> ()
          }
          frame #3 {
            n205 = global read "Global.vi" "Result"() -> (w411:refnum<vi>)
            n206 = global read "Global1.vi" "用户信息"() -> (w401:T5)
            n207 = property class="Tbl"(reference=w411, "Row Headers[]"=string[] [], "Value"=string[][] []) -> ()  [unwired: 1 in, 2 out]
            n208 = Unbundle By Name(w401) -> ("用户名"=w402:string)
            n209 = vi-ref "client.vi"() -> (w399:refnum<vi>)
            n210 = Bundle("设备名称"="滑移力检测", "用户名"=w402, "设备状态"=enum16{"设备离线", "设备正常", "设备缺料", "设备故障", "质量报警"}."设备正常", "附加信息"="") -> (w403:T8)  [unwired: 1 in]
            n211 = invoke class="VI" method="Ctrl Val.Set"(reference=w399, "Control Name"="设备信息" ("控件名"), "Value"=w403) -> (reference out=w400:refnum<vi>)  [unwired: 2 in, 4 out]
            n212 = call "CallVI.vi"("VI引用"=w400, "状态"=T2."Hidden") -> ()  [unwired: 12 in, 2 out]
          }
        }
        n213 = call <vilib>:"Add State(s) to Queue__jki_lib_state_machine.vi"("State(s) in (\"\")"=w378) -> ("States Out"=w377:string)  [unwired: 14 in]
      }
      frame "UI: Config" {
        n214 = call <vilib>:"Add State(s) to Queue__jki_lib_state_machine.vi"("State(s) in (\"\")"=w417) -> ("States Out"=w416:string)  [unwired: 14 in]
      }
      frame "UI: Cursor Set" {
        # "Argument"
        n215 = case shown="\"Idle\", 默认" w420 {
          tunnel: w422 -> [w427 w429]
          tunnel: [w426 w428] -> w421
          frame "Idle", Default {
            n216 = call <vilib>:"Unset Busy.vi"("error in (no error)"=w427) -> ("error out"=w426:errorcluster)  [unwired: 10 in]
          }
          frame "Busy" {
            n217 = call <vilib>:"Set Busy.vi"("error in (no error)"=w429) -> ("error out"=w428:errorcluster)  [unwired: 9 in, 1 out]
          }
        }
        n218 = call <vilib>:"Add State(s) to Queue__jki_lib_state_machine.vi"("State(s) in (\"\")"=w425) -> ("States Out"=w424:string)  [unwired: 14 in]
      }
      frame "UI: Front Panel State" {
        # "Argument"
        n219 = Unbundle By Name(w434) -> ("Core.Current VI Reference"=w433:refnum<vi>)
        n220 = case shown="\"Open\", 默认" w432 {
          tunnel: w436 -> [w442 w455]
          tunnel: [w444 w456] -> w435
          tunnel: w433 -> [w443 w453]
          frame "Open", Default {
            n221 = property class="VI"(reference=w443, error in=w442) -> (reference out=w440:refnum<vi>, error out=w441:errorcluster, "Front Panel.Open"=w439:bool)
            n222 = case shown="假" w439 {
              tunnel: [w447 w450] -> w444
              tunnel: w441 -> [w446 w450]
              tunnel: w440 -> [w445 _]
              frame False {
                n223 = invoke class="VI" method="FP.Open"(reference=w445, error in=w446, "Activate"=TRUE, "State"=T2."Standard") -> (error out=w447:errorcluster)  [unwired: 1 in, 4 out]
              }
              frame True {
              }
            }
          }
          frame "Close" {
            n224 = property class="VI"(reference=w453, error in=w455) -> (reference out=w452:refnum<vi>, error out=w454:errorcluster, "Front Panel.Open"=w451:bool)
            n225 = case shown="真" w451 {
              tunnel: [w457 w460] -> w456
              tunnel: w454 -> [w457 w459]
              tunnel: w452 -> [_ w458]
              frame False {
              }
              frame True {
                n226 = invoke class="VI" method="FP.Close"(reference=w458, error in=w459) -> (error out=w460:errorcluster)  [unwired: 1 in, 2 out]
              }
            }
          }
        }
        n227 = call <vilib>:"Add State(s) to Queue__jki_lib_state_machine.vi"("State(s) in (\"\")"=w438) -> ("States Out"=w437:string)  [unwired: 14 in]
      }
      frame "---------- Macro ----------" {
        n228 = call <vilib>:"Add State(s) to Queue__jki_lib_state_machine.vi"("State(s) in (\"\")"=w466) -> ("States Out"=w465:string)  [unwired: 14 in]
      }
      frame "Macro: Initialize" {
        n229 = call <vilib>:"Add State(s) to Queue__jki_lib_state_machine.vi"("State(s) in Front (\"\")"="Data: Initialize\nInitialize Core Data\nS7: Initialize\nIdle\nUI: Init\nUI: Front Panel State >> Open\nUI: Initialize\nUI: Config", "State(s) in (\"\")"=w473) -> ("States Out"=w472:string)  [unwired: 13 in]
      }
      frame "Macro: Exit" {
        n230 = Unbundle By Name(w482) -> ("Core.Close Panel on Exit?"=w481:bool)
        n231 = Select(t="UI: Front Panel State >> Close", s=w481, f="") -> (s? t:f=w478:string)
        n232 = call <vilib>:"Add State(s) to Queue__jki_lib_state_machine.vi"("State(s) in (\"\")"=w478, "State(s) at Back (\"\")"="Data: Cleanup\nExit") -> ("States Out"=w476:string)  [unwired: 13 in]
        n233 = call <vilib>:"Add State(s) to Queue__jki_lib_state_machine.vi"("State(s) in Front (\"\")"=w476, "State(s) in (\"\")"=w485) -> ("States Out"=w484:string)  [unwired: 13 in]
      }
    }
  }
  n234 = call-dynamic "Cleanup.vi"("MenuStrip in"=w6) -> ()  [unwired: 10 in, 1 out]
